vi "Measure DC 120629.vi"() -> ()   [LabVIEW 2011]
uses:
  Sub VIs/Trap cluster.ctl
  <vilib>/Utility/inputDevices.llb/closeKeyboard.vi
  <vilib>/Utility/inputDevices.llb/keyboardAcquire.vi
  <vilib>/Utility/file.llb/Write To Spreadsheet File (I64).vi
  <vilib>/vision/driver/NI_Vision_Acquisition_Software.lvlib
  <vilib>/vision/NI_Vision_Development_Module.lvlib
panel:
  in  "Apply Corrections":bool
  in  "View Licence":bool
  in  "ok":bool caption="Mark the center of \nthe spot using the \nzoom and the point\ntool, then click this \nbutton"
  in  "Stop program":bool
  in  "Updating trap cluster":bool
  out "Camera enabled":bool=TRUE
  out "SLM enabled":bool=TRUE
  in  "Run calibration":bool
  in  "Hologram generation":cluster{"Method":i32, "Iterations":i32}={"Method"=1, "Iterations"=50} {"Method" items=["Lenses & Gratings (3D)", " Gerchberg-Saxton (3D)", "Gerchberg-Saxton FFT (2D)"]}
  in  "Display hologram\nand computed \nimage plane":bool
  in  "ROI":T1={"Global Rectangle"=[39, 191, 388, 192], "Contours"=[{"Contour Type"=0, "ROI Type"=1, "Points"=[387, 191]}, {"Contour Type"=0, "ROI Type"=1, "Points"=[300, 191]}, {"Contour Type"=0, "ROI Type"=1, "Points"=[213, 191]}, {"Contour Type"=0, "ROI Type"=1, "Points"=[126, 191]}, {"Contour Type"=0, "ROI Type"=1, "Points"=[39, 191]}]}
  out "Image":T2(plugin-control)
  in  "Save\nHologram":bool
  in  "Image\naveraging":i32=100
  in  "?":bool
  in  "?":bool
  out "e desired":sgl=25.0
  out "timed out?":bool
  in  "Sync \nmeasurement":bool
  in  "images per \nhologram":i32=1
  in  "I step":dbl=0.05
  in  "Intensity path":bool
  in  "?":bool=TRUE
  out "Global Report":T3={"Mean Value"=0.014534721, "Standard Variation"=0.33891603, "Minimal Value"=0.0, "Maximal Value"=57.52, "Area (calibrated)"=1310720.0, "Area (pixels)"=1310720, "%"=100.0, "Calibration Valid"=TRUE} {"Mean Value" format="%.2f"; "%" format="%.2f"; "Area (calibrated)" format="%.2f"; "Maximal Value" format="%.2f"; "Minimal Value" format="%.2f"; "Standard Variation" format="%.2f"}
  in  "start path":path=path "E:/David/SLM characterization/Measured data/120420 - Trapping"
  in  "?":bool
  in  "s":bool=TRUE
  in  "Edit trap cluster":bool
  out "Lost Frames":u32
  in  "threshold":bool
  in  "Range":cluster{"Lower value":sgl, "Upper value":sgl}={"Lower value"=200.0, "Upper value"=4096.0} {"Upper value" format="%.2f"; "Lower value" format="%.2f"}
  in  "Display data":bool=TRUE
  in  "?":bool=TRUE
  in  "Purge data":bool
  in  "ROI size":dbl=44.0 min=2.0 step=2.0
  in  "Save data":bool
  in  "Video tracking":bool
  out "Calculated image plane":dbl[][](graph)
  out "Current trap pos":T4={"X (IMAQ)"=[451.25, 557.0, 662.75, 821.375, 874.25, 980.0, 1085.75], "Y (IMAQ)"=[588.5, 588.5, 588.5, 740.5156, 588.5, 588.5, 588.5], "Z"=[0.0, 0.0, 0.0, 0.0, 0.0, 0.0, 0.0], "I"=[0.0, 0.0, 0.0, 100.0, 100.0, 100.0, 0.0], "Trap number"=[0, 1, 2, 3, 4, 5, 6], "ROI number"=[0, 1, 2, 3, 4, 5, 6], "Number of traps"=7, "Group"=[FALSE, FALSE, FALSE, FALSE, FALSE, FALSE, FALSE]}
  out "NI Vision error":errorcluster
  out "CUDA/SLM error":errorcluster
  in  "Cancel calibration":bool
  in  "Skip step if \ntimed out":bool
  in  "Display path":bool=TRUE
  out "Average step time (ms)":dbl=61.852387843704776
  in  "Step time \n(ms)":u32=10
  in  "Pause":bool
  in  "cancel path":bool
  out "Step skipped":bool
  in  "Path controls":T5={"follow path"=FALSE, "Step length"=1.0, "Arrive \nsimultaneously"=TRUE, "Synchronize traps"=FALSE, "Add current \npositions to path"=FALSE}
  in  "Create path":bool
  out "Displayed Hologram":u8[][](graph)
  in  "Coordinate mapping \n(IMAQ to SLM)":T6={"cZ"=1.0, "cY"=0.3699422, "cX"=-0.3699422, "sZ"=0.0, "sY"=-181.0867, "sX"=244.71677}
  in  "Switch X/Y":bool
  in  "Max num of \nmeasurements":i32=-1
  # "Martin\nPersson 2011"
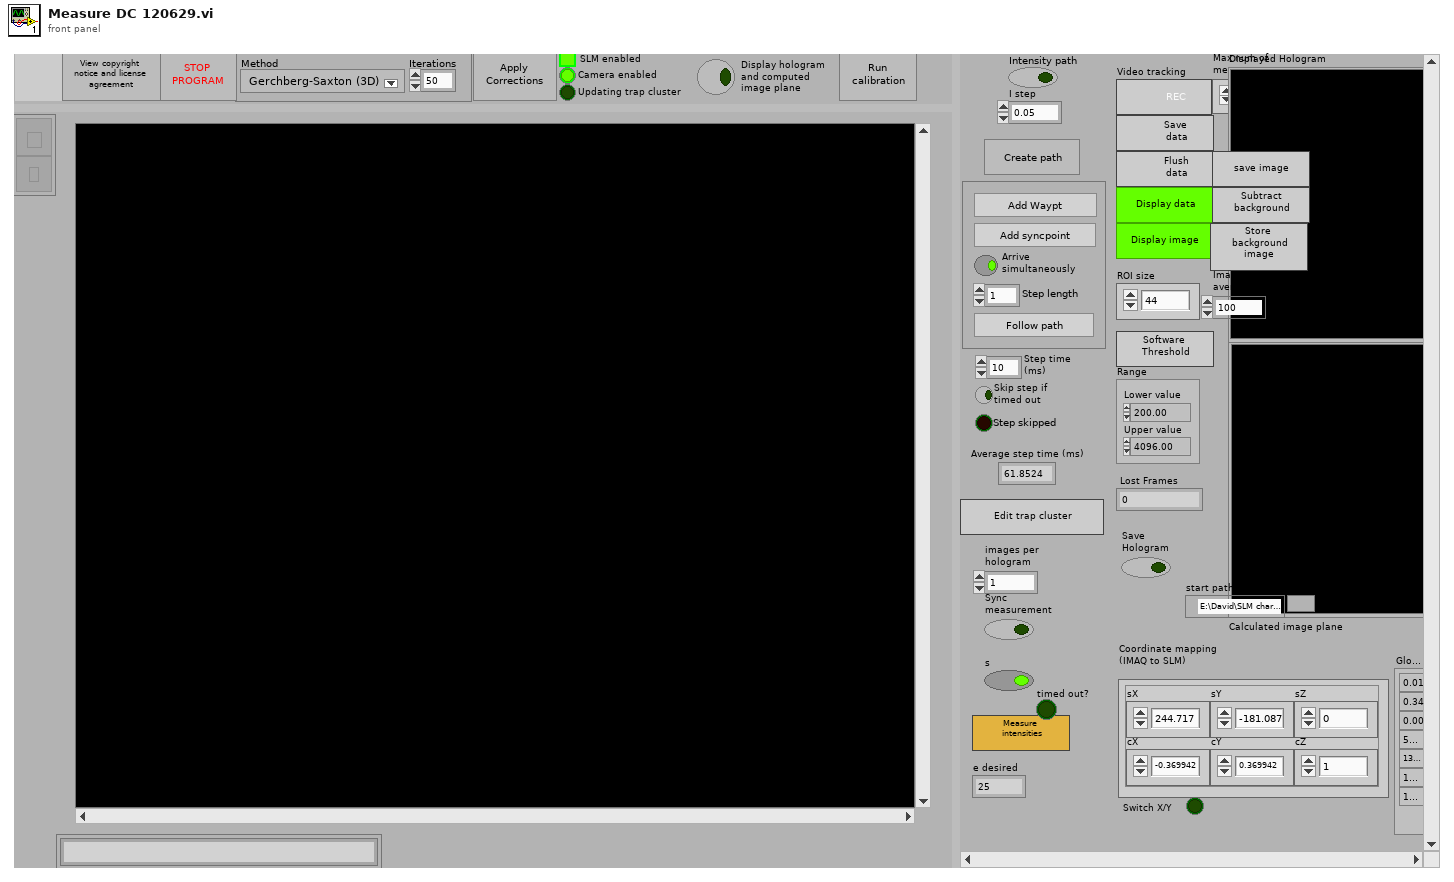
[diagram p1: front panel]
types:
  T1 = cluster{"Global Rectangle":i32[], "Contours":cluster{"Contour Type":u32, "ROI Type":u32, "Points":i32[]}[]}
  T2 = typedef "IMAQ Image.ctl" = refnum<image>
  T3 = cluster{"Mean Value":sgl, "Standard Variation":sgl, "Minimal Value":sgl, "Maximal Value":sgl, "Area (calibrated)":sgl, "Area (pixels)":u32, "%":sgl, "Calibration Valid":bool}
  T4 = typedef "Trap cluster.ctl" = cluster{"X (IMAQ)":sgl[], "Y (IMAQ)":sgl[], "Z":sgl[], "I":sgl[], "Trap number":i32[], "ROI number":i32[], "Number of traps":i32, "Group":bool[]}
  T5 = cluster{"follow path":bool, "Step length":dbl, "Arrive \nsimultaneously":bool, "Synchronize traps":bool, "Add current \npositions to path":bool}
  T6 = cluster{"cZ":sgl, "cY":sgl, "cX":sgl, "sZ":sgl, "sY":sgl, "sX":sgl}
  T7 = typedef "Image Type" = u32
  T8 = cluster{"CentroidX":dbl[], "CentroidY":dbl[], "I":dbl[], "Acquired Buffer Number":u32}
  T9 = typedef "IMAQdx.ctl" = refnum<k21>
  T10 = typedef "Rendezvous RefNum" = refnum<k1>
  T11 = enum16{"0", "1", "2", "3", "4", "5", "6", "7", "8", "9", "A", "B", "C", "D", "E", "F", "G", "H", "I", "J", "K", "L", "M", "N", "O", "P", "Q", "R", "S", "T", "U", "V", "W", "X", "Y", "Z", "F1", "F2", "F3", "F4", "F5", "F6", "F7", "F8", "F9", "F10", "F11", "F12", "F13", "F14", "F15", "ADD", "BACK", "BACKSLASH", "CAPITAL", "COMMA", "DECIMAL", "DELETE", "DIVIDE", "DOWN", "END", "EQUALS", "ESCAPE", "GRAVE (`)", "HOME", "INSERT", "LBRACKET", "LCONTROL", "LEFT", "L ALT", "LSHIFT", "LWIN", "MINUS", "MULTIPLY", "NEXT", "NUMLOCK", "NUMPAD_0", "NUMPAD_1", "NUMPAD_2", "NUMPAD_3", "NUMPAD_4", "NUMPAD_5", "NUMPAD_6", "NUMPAD_7", "NUMPAD_8", "NUMPAD_9", "PAUSE", "PERIOD", "PRIOR (PG UP)", "RBRACKET", "RCONTROL", "RETURN", "RIGHT", "R ALT", "RSHIFT", "RWIN", "SCROLL", "SEMICOLON", "SLASH", "SPACE", "SUBTRACT", "TAB", "UP", "ENTER (num pad)", "' (quote)"}[]
  T12 = typedef "LVRectTypeDef.ctl" = cluster{"left":i16, "top":i16, "right":i16, "bottom":i16}
  T13 = cluster{"output cluster 2":cluster{"CentroidX":dbl[], "CentroidY":dbl[], "I":dbl[], "Acquired Buffer Number":u32}, "output cluster 2":T4}[]
  T14 = cluster{"CentroidX":dbl[], "CentroidY":dbl[], "I":dbl[], "Acquired Buffer Number":u32}[]
  T15 = cluster{"output cluster 2":cluster{"CentroidX":dbl[], "CentroidY":dbl[], "I":dbl[], "Acquired Buffer Number":u32}, "output cluster 2":T4}
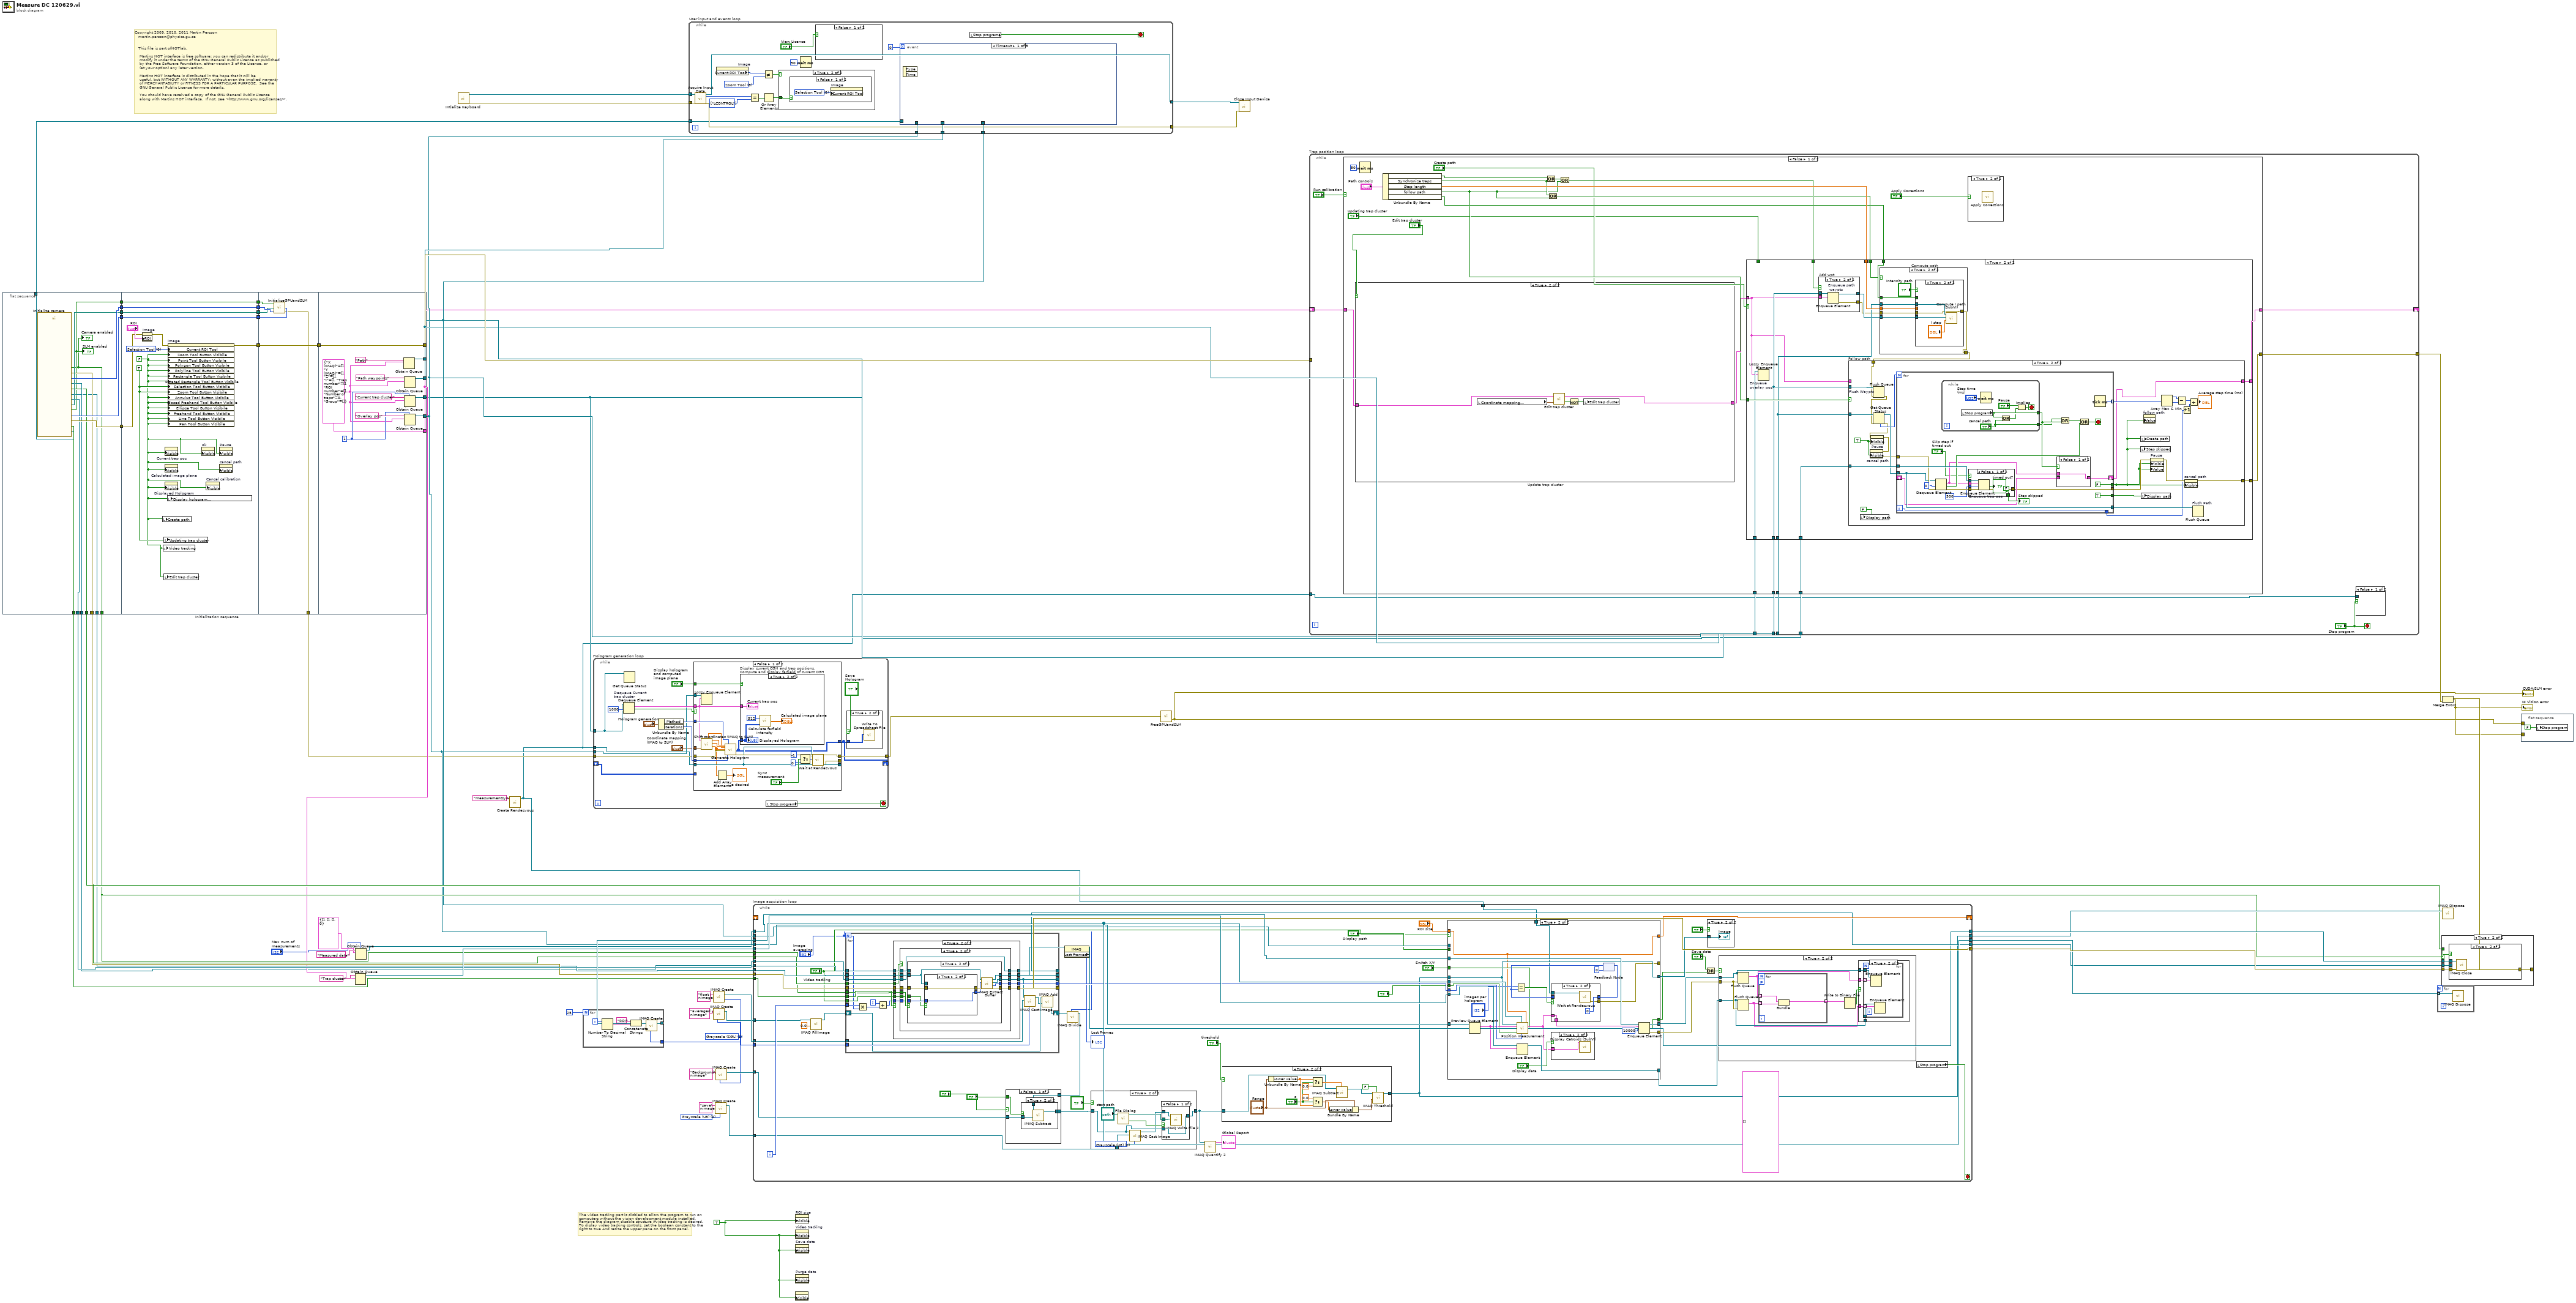
[diagram p0: block diagram]
diagram:
  w2 = T7 0 items=["Grayscale (U8)", "Grayscale (I16)", "Grayscale (SGL)", "Complex (CSG)", "RGB (U32)", "HSL (U32)", "RGB (U64)", "Grayscale (U16)"] ("Image Type")
  w4 = T7 2 items=["Grayscale (U8)", "Grayscale (I16)", "Grayscale (SGL)", "Complex (CSG)", "RGB (U32)", "HSL (U32)", "RGB (U64)", "Grayscale (U16)"] ("Image Type")
  w49 = TRUE ("Visible")
  # "Copyright 2009, 2010, 2011 Martin Persson \n   martin.persson@physics.gu.se\n\n\n   This file is part ofHOTlab.\n\n    Martins HOT interface is free software: you can redistribute it and/or \n    modify it under the terms of the GNU General Public License as published \n    by the Free Software Foundation, either version 3 of the License, or\n    (at your option) any later version.\n\n    Martins HOT interface is distributed in the hope that it will be \n    useful, but WITHOUT ANY WARRANTY; without even the implied warranty\n    of MERCHANTABILITY or FITNESS FOR A PARTICULAR PURPOSE.  See the\n    GNU General Public License for more details.\n\n    You should have received a copy of the GNU General Public License\n    along with Martins HOT interface.  If not, see <http://www.gnu.org/licenses/>."
  # "The video tracking part is disbled to allow the program to run on\ncomputers without the vision development module installed. \nRemove the diagram disable structure ifvideo tracking is desired. \nTo diplay video tracking controls, set the boolean constant to the \nright to true And resize the upper pane on the front panel."
  n1 = flat-sequence "Initialization sequence" {
    tunnel: [w65] -> w41
    tunnel: [w74] -> w40
    tunnel: [w73] -> w39
    tunnel: [w72] -> w38
    tunnel: [w71] -> w37
    tunnel: [w70] -> w17
    tunnel: [w69] -> w35
    tunnel: [w68] -> w34
    tunnel: [w67] -> w33
    tunnel: [w66] -> w32
    tunnel: [w64] -> w31
    tunnel: [w63] -> w18
    tunnel: [w62] -> w16
    tunnel: w41 -> [w82]
    tunnel: w40 -> [w80]
    tunnel: w39 -> [w85]
    tunnel: w38 -> [w84]
    tunnel: w37 -> [w83]
    tunnel: [w82] -> w26
    tunnel: [w77] -> w25
    tunnel: [w85] -> w23
    tunnel: [w84] -> w22
    tunnel: [w83] -> w21
    tunnel: w26 -> [w88]
    tunnel: w25 -> [w91]
    tunnel: [w91] -> w24
    tunnel: w23 -> [w89]
    tunnel: w22 -> [w90]
    tunnel: w21 -> [w87]
    tunnel: [w86] -> w20
    tunnel: [w102] -> w36
    tunnel: w24 -> [w102]
    tunnel: [w100] -> w30
    tunnel: [w98] -> w29
    tunnel: [w96] -> w19
    tunnel: [w95] -> w28
    tunnel: [w92] -> w27
    frame #0 {
      n2 = call "Initialize camera.vi"() -> ("CUDA device ID"=w72:i32, "IMAQdx Session Out"=w69:T9, "TrueFrame out"=w73:i32, "IMAQ camera"=w67:bool, "Image buffers"=w62:T2[], "Image reference out"=w70:T2, "Ring?"=w63:bool, "SLM enabled"=w65:bool, "Camera enabled"=w64:bool, "Vision error out"=w74:errorcluster, "LUT path out"=w71:path, "IMAQ Session Out"=w66:refnum<k11>, "Camera error"=w68:errorcluster)  [unwired: 3 in]
      "Camera enabled" <- w64
      "SLM enabled" <- w65
    }
    frame #1 {
      w76 = TRUE ("ROI Tool Buttons Visibile:Zoom Tool Button Visible")
      w75 = FALSE ("ROI Tool Buttons Visibile:Zoom Tool Button Visible")
      w79 = u32 0 items=["Zoom Tool"=8, "Selection Tool"=0, "Pan Tool"=9, "Point Tool"=1, "Line Tool"=2, "Rectangle Tool"=3, "Rotated Rectangle Tool"=12, "Polyline Tool"=10, "Polygon Tool"=5, "Freehand Tool"=11, "Closed Freehand Tool"=6, "Ellipse Tool"=4, "Annulus Tool"=7] ("Current ROI Tool")
      n3 = property on="Image" class="ImageControl"(error in=w80, "ROI"="ROI") -> (error out=w78:errorcluster)  [unwired: 1 in, 1 out]
      n4 = local write "Create path"(w75) -> ()
      n5 = local write "Video tracking"(w75) -> ()
      n6 = local write "Updating trap cluster"(w76) -> ()
      n7 = local write "Edit trap cluster"(w75) -> ()
      n8 = property on="Current trap pos" class="Clust (strict)"("Visible"=w75) -> ()  [unwired: 2 in, 2 out]
      n9 = property on="Calculated image plane" class="IntGraph (strict)"("Visible"=w75) -> ()  [unwired: 2 in, 2 out]
      n10 = property on="Displayed Hologram" class="IntGraph (strict)"("Visible"=w75) -> ()  [unwired: 2 in, 2 out]
      n11 = local write "Display hologram\nand computed \nimage plane"(w75) -> ()
      n12 = property on="Image" class="ImageControl"(error in=w78, "Current ROI Tool"=w79, "Zoom Tool Button Visibile"=w75, "Point Tool Button Visibile"=w75, "Polygon Tool Button Visibile"=w75, "Polyline Tool Button Visibile"=w75, "Rectangle Tool Button Visibile"=w75, "Rotated Rectangle Tool Button Visibile"=w75, "Selection Tool Button Visibile"=w76, "Zoom Tool Button Visibile"=w76, "Annulus Tool Button Visibile"=w75, "Closed Freehand Tool Button Visibile"=w75, "Ellipse Tool Button Visibile"=w75, "Freehand Tool Button Visibile"=w75, "Line Tool Button Visibile"=w75, "Pan Tool Button Visibile"=w75) -> (error out=w77:errorcluster)  [unwired: 1 in, 1 out]
      n13 = property on="ok" class="Bool"("Visible"=w75) -> ()  [unwired: 2 in, 2 out]
      n14 = property on="Cancel calibration" class="Bool"("Visible"=w75) -> ()  [unwired: 2 in, 2 out]
      n15 = property on="Pause" class="Bool (strict)"("Visible"=w75) -> ()  [unwired: 2 in, 2 out]
      n16 = property on="cancel path" class="Bool"("Visible"=w75) -> ()  [unwired: 2 in, 2 out]
    }
    frame #2 {
      n17 = call "InitializeGPUandSLM.vi"("TrueFrame"=w89, "deviceId"=w90, "Path to LUT file"=w87, "SLM enabled"=w88) -> ("CUDA/SLM error"=w86:errorcluster)  [unwired: 1 out]
    }
    frame #3 {
      w93 = 1 ("max queue size (-1, unlimited)")
      w92 = T4 {"X (IMAQ)"=[], "Y (IMAQ)"=[], "Z"=[], "I"=[], "Trap number"=[], "ROI number"=[], "Number of traps"=0, "Group"=[]} ("output cluster 2")
      n18 = Obtain Queue(name (unnamed)="Path", element data type=w92) -> (queue out=w100:refnum<queue>)  [unwired: 3 in, 2 out]
      n19 = Obtain Queue(name (unnamed)="Path waypoints", element data type=w92) -> (queue out=w98:refnum<queue>)  [unwired: 3 in, 2 out]
      n20 = Obtain Queue(max queue size (-1, unlimited)=w93, name (unnamed)="Current trap cluster", element data type=w92) -> (queue out=w96:refnum<queue>)  [unwired: 2 in, 2 out]
      n21 = Obtain Queue(max queue size (-1, unlimited)=w93, name (unnamed)="Overlay pos", element data type=w92) -> (queue out=w95:refnum<queue>)  [unwired: 2 in, 2 out]
    }
  }
  n22 = Obtain Queue(name (unnamed)="Trap cluster", element data type=w27) -> (queue out=w54:refnum<queue>)  [unwired: 3 in, 2 out]
  n23 = Obtain Queue(max queue size (-1, unlimited)="Max num of \nmeasurements", name (unnamed)="Measured data", element data type=T8 {"CentroidX"=[], "CentroidY"=[], "I"=[], "Acquired Buffer Number"=0} ("output cluster 2")) -> (queue out=w13:refnum<queue>)  [unwired: 2 in, 2 out]
  n24 = call <vilib>:"Intialize Keyboard.vi"() -> ("error out"=w43:errorcluster, "device ID"=w61:refnum<k1>)  [unwired: 1 in, 9 out]
  n25 = call <vilib>:"Create Rendezvous.vi"("name (unnamed)"="measurementsync") -> ("rendezvous"=w11:T10)  [unwired: 4 in, 2 out]
  n26 = for {
    N: 25 -> [_]
    tunnel: [w108] -> w58 mode=indexing
    tunnel: w4 -> [w103]
    i -> [w105]
    n27 = Number To Decimal String(number=w105) -> (decimal integer string=w104:string)  [unwired: 1 in]
    n28 = Concatenate Strings("ROI" ("Image Name"), w104) -> (w106:string)
    n29 = call "IMAQ Create"("Image Name"=w106, "Image Type"=w103) -> ("New Image"=w108:T2)  [unwired: 3 in, 1 out]
  }
  n30 = while "Hologram generation loop" {
    tunnel: w19 -> [w112]
    tunnel: w28 -> [w121]
    tunnel: w20 -> [w116]
    tunnel: [w115] -> w14
    tunnel: w11 -> [w114]
    shift-right: [w111] -> _
    shift-left: _ -> [w110]
    stop <- w113 stop-if-true
    n31 = Dequeue Element "Dequeue Current \ntrap cluster"(queue=w112, timeout in ms (-1)=1000) -> (element=w122:T4, timed out?=w120:bool)  [unwired: 1 in, 2 out]
    n32 = Get Queue Status(queue=w112) -> ()  [unwired: 2 in, 8 out]
    n33 = Unbundle By Name("Hologram generation") -> ("Method"=w125:i32, "Iterations"=w124:i32)
    n34 = case shown="False" w120 {
      tunnel: "Coordinate mapping \n(IMAQ to SLM)" -> [w146 _]
      tunnel: "Display hologram\nand computed \nimage plane" -> [w139 _]
      tunnel: w125 -> [w142 _]
      tunnel: w124 -> [w141 _]
      tunnel: w122 -> [w136 _]
      tunnel: w121 -> [w140 _]
      tunnel: w116 -> [w138 w153]
      tunnel: [w137 w153] -> w115
      tunnel: w114 -> [w131 w152]
      tunnel: [w131 w152] -> _
      tunnel: [w130 _] -> _
      tunnel: [w127 w151] -> w111
      tunnel: w110 -> [_ w151]
      frame False {
        n35 = Lossy Enqueue Element(queue=w140, element=w136) -> ()  [unwired: 1 in, 4 out]
        n36 = call "Shift coordinates (IMAQ to SLM).vi"("Trap cluster"=w136, "Coordinate mapping \n(IMAQ to SLM)"=w146) -> ("X (SLM)"=w143:sgl[], "Y (SLM)"=w145:sgl[], "Intensities"=w129:sgl[], "Z (SLM)"=w144:sgl[])  [unwired: 1 in, 1 out]
        n37 = Add Array Elements(numeric array=w129) -> (sum=→"e desired":sgl)
        n38 = call "Generate Hologram.vi"("x"=w143, "y"=w145, "z"=w144, "spot_intensities"=w129, "CUDA/SLM error in"=w138, "N_iterations"=w141, "method"=w142) -> ("CGH out"=w127:u8[][], "CUDA/SLM error out"=w137:errorcluster)  [unwired: 17 in, 2 out]
        n39 = case "Display current CGH and trap positions.\nCompute and display farfield of current CGH" shown="True" w139 {
          tunnel: w127 -> [_ w149]
          tunnel: w136 -> [_ w147]
          frame False {
          }
          frame True {
            n40 = call "Calculate farfield intensity.vi"("h_pSLM"=w149, "SLMsize"=512 ("Numeric")) -> ("Calculated image plane"=→"Calculated image plane":dbl[][])
            "Displayed Hologram" <- w149
            "Current trap pos" <- w147
          }
        }
        n41 = Select(t=-1 ("ms timeout (-1)"), s="Sync \nmeasurement", f=0) -> (s? t:f=w133:i32)
        n42 = call <vilib>:"Wait at Rendezvous.vi"("ms timeout (-1)"=w133, "rendezvous"=w131) -> ("error out"=w130:errorcluster)  [unwired: 3 in, 2 out]
      }
      frame True {
      }
    }
    n43 = local read "Stop program"() -> (w113:bool)
    n44 = case shown="True" "Save\nHologram" {
      tunnel: w111 -> [_ w126]
      frame False {
      }
      frame True {
        n45 = call-poly <vilib>:"Write To Spreadsheet File.vi"("2D data"=w126) -> ()  [unwired: 7 in, 1 out]
      }
    }
  }
  n46 = while "User input and events loop" {
    tunnel: w61 -> [w172]
    tunnel: w28 -> [w161]
    tunnel: w29 -> [w160]
    tunnel: w30 -> [w159]
    tunnel: [w158] -> w44
    tunnel: w43 -> [w157]
    tunnel: [w156] -> w42
    tunnel: w16 -> [w154]
    stop <- w164 stop-if-true
    w169 = u32 8 items=["Zoom Tool"=8, "Selection Tool"=0, "Pan Tool"=9, "Point Tool"=1, "Line Tool"=2, "Rectangle Tool"=3, "Rotated Rectangle Tool"=12, "Polyline Tool"=10, "Polygon Tool"=5, "Freehand Tool"=11, "Closed Freehand Tool"=6, "Ellipse Tool"=4, "Annulus Tool"=7] ("Current ROI Tool")
    w166 = T11 [enum."LCONTROL"] items=["0", "1", "2", "3", "4", "5", "6", "7", "8", "9", "A", "B", "C", "D", "E", "F", "G", "H", "I", "J", "K", "L", "M", "N", "O", "P", "Q", "R", "S", "T", "U", "V", "W", "X", "Y", "Z", "F1", "F2", "F3", "F4", "F5", "F6", "F7", "F8", "F9", "F10", "F11", "F12", "F13", "F14", "F15", "ADD", "BACK", "BACKSLASH", "CAPITAL", "COMMA", "DECIMAL", "DELETE", "DIVIDE", "DOWN", "END", "EQUALS", "ESCAPE", "GRAVE (`)", "HOME", "INSERT", "LBRACKET", "LCONTROL", "LEFT", "L ALT", "LSHIFT", "LWIN", "MINUS", "MULTIPLY", "NEXT", "NUMLOCK", "NUMPAD_0", "NUMPAD_1", "NUMPAD_2", "NUMPAD_3", "NUMPAD_4", "NUMPAD_5", "NUMPAD_6", "NUMPAD_7", "NUMPAD_8", "NUMPAD_9", "PAUSE", "PERIOD", "PRIOR (PG UP)", "RBRACKET", "RCONTROL", "RETURN", "RIGHT", "R ALT", "RSHIFT", "RWIN", "SCROLL", "SEMICOLON", "SLASH", "SPACE", "SUBTRACT", "TAB", "UP", "ENTER (num pad)", "' (quote)"] ("keys pressed")
    n47 = call-poly <vilib>:"Acquire Input Data.vi"("device ID"=w172, "error in (no error)"=w157) -> ("device ID"=w158:refnum<k1>, "keys pressed"=w165:T11, "error out"=w156:errorcluster)  [unwired: 15 out]
    n48 = property on="Image" class="ImageControl"() -> ("Current ROI Tool"=w168:u32)  [unwired: 2 in, 2 out]
    n49 = Equal?(x=w165, y=w166) -> (x = y?=w167:bool[])
    n50 = Not Equal?(x=w168, y=w169) -> (x != y?=w170:bool)
    n51 = Or Array Elements(Boolean array=w167) -> (logical OR=w171:bool)
    n52 = case shown="True" w170 {
      tunnel: w171 -> [_ w206]
      frame False {
      }
      frame True {
        n53 = case shown="False" w206 {
          frame False {
            w207 = u32 0 items=["Zoom Tool"=8, "Selection Tool"=0, "Pan Tool"=9, "Point Tool"=1, "Line Tool"=2, "Rectangle Tool"=3, "Rotated Rectangle Tool"=12, "Polyline Tool"=10, "Polygon Tool"=5, "Freehand Tool"=11, "Closed Freehand Tool"=6, "Ellipse Tool"=4, "Annulus Tool"=7] ("Current ROI Tool")
            n54 = property on="Image" class="ImageControl"("Current ROI Tool"=w207) -> ()  [unwired: 2 in, 2 out]
          }
          frame True {
            w208 = u32 1 items=["Zoom Tool"=8, "Selection Tool"=0, "Pan Tool"=9, "Point Tool"=1, "Line Tool"=2, "Rectangle Tool"=3, "Rotated Rectangle Tool"=12, "Polyline Tool"=10, "Polygon Tool"=5, "Freehand Tool"=11, "Closed Freehand Tool"=6, "Ellipse Tool"=4, "Annulus Tool"=7] ("Current ROI Tool")
            n55 = property on="Image" class="ImageControl"("Current ROI Tool"=w208) -> ()  [unwired: 2 in, 2 out]
          }
        }
      }
    }
    n56 = Wait (ms)(milliseconds to wait=u32 50) -> ()  [unwired: 1 out]
    n57 = case shown="False" "View Licence" {
      frame False {
      }
      frame True {
        n58 = call "View license.vi"() -> ()  [unwired: 1 in]
      }
    }
    n59 = event shown="[0] Timeout" {
      selector: _ -> [_ _ _ _ _ _ _ _ _]
      dyn-events: _ -> [_ _ _ _ _ _ _ _ _]
      timeout: 0 -> [_ _ _ _ _ _ _ _ _]
      tunnel: w161 -> [_ _ w183 _ _ _ _ _ _]
      tunnel: w160 -> [_ _ w182 _ _ _ _ _ _]
      tunnel: w159 -> [_ _ w186 _ _ _ _ _ _]
      tunnel: w154 -> [_ _ _ _ _ _ w198 _ _]
      event Timeout {
        n60 = event-data() -> ()  [unwired: 1 in, 2 out]
      }
      event "Display hologram\nand computed \nimage plane": Value Change {
        n61 = event-data() -> ("NewVal"=w174:bool)  [unwired: 1 in, 4 out]
        n62 = property on="Current trap pos" class="Clust (strict)"("Visible"=w174) -> ()  [unwired: 2 in, 2 out]
        n63 = property on="Displayed Hologram" class="IntGraph (strict)"("Visible"=w174) -> ()  [unwired: 2 in, 2 out]
        n64 = property on="Calculated image plane" class="IntGraph (strict)"("Visible"=w174) -> ()  [unwired: 2 in, 2 out]
        n65 = property on="Property Node" class="VI"() -> ("Front Panel.WinBounds"=w181:T12)  [unwired: 2 in, 2 out]
        n66 = Unbundle By Name(w181) -> ("right"=w180:i16, "left"=w179:i16)
        n67 = Subtract(x=w180, y=w179) -> (x-y=w178:i16)
        n68 = Select(t=i16 500 ("x-y"), s=w174, f=i16 196 ("x-y")) -> (s? t:f=w173:i16)
        n69 = Subtract(x=w178, y=w173) -> (x-y=w177:i16)
        n70 = property on="Splitter" class="Splitter"("Position"=w177) -> ()  [unwired: 2 in, 2 out]
      }
      event "Create path": Value Change {
        n71 = event-data() -> ()  [unwired: 1 in, 5 out]
        n72 = property on="follow path" class="Bool (strict)"("Value"=FALSE) -> ()  [unwired: 2 in, 2 out]
        n73 = Flush Queue "Flush path \nwaypt queue"(queue=w182) -> ()  [unwired: 1 in, 3 out]
        n74 = Preview Queue Element(queue=w183) -> (element=w184:T4, error out=w187:errorcluster)  [unwired: 2 in, 2 out]
        n75 = Flush Queue "Flush path queue"(queue=w186) -> (queue out=w185:refnum<queue>)  [unwired: 1 in, 2 out]
        n76 = Enqueue Element "Enqueue current \ntrap pos in path"(queue=w185, element=w184) -> ()  [unwired: 2 in, 3 out]
        n77 = Enqueue Element "Enqueue current \ntrap pos in path \nwaypts"(queue=w182, element=w184, error in (no error)=w187) -> ()  [unwired: 1 in, 3 out]
      }
      event "cancel path": Value Change {
        n78 = event-data() -> ()  [unwired: 1 in, 5 out]
        n79 = local write "Create path"(FALSE ("Visible")) -> ()
      }
      event "Image", "Coordinate mapping \n(IMAQ to SLM)": Mouse Down {
        w190 = FALSE ("Edit trap cluster")
        n80 = event-data() -> ()  [unwired: 1 in, 7 out]
        n81 = local write "Updating trap cluster"(TRUE ("Update trap positions")) -> ()
        n82 = local write "Edit trap cluster"(w190) -> ()
        n83 = call <vilib>:"Application Directory.vi"() -> ("Application Directory"=w191:path)
        n84 = Build Path(base path=w191, name or relative path="Sub VIs\\Edit trap cluster.vi") -> (appended path=w194:path)
        n85 = Open VI Reference(vi path=w194) -> (vi reference=w193:refnum<vi>)  [unwired: 5 in, 1 out]
        n86 = property class="VI"(reference=w193, "Front Panel.Open"=w190) -> ()  [unwired: 1 in, 2 out]
      }
      event "Image", "Coordinate mapping \n(IMAQ to SLM)": Mouse Up {
        n87 = event-data() -> ()  [unwired: 1 in, 7 out]
        n88 = flat-sequence {
          frame #0 {
            n89 = Wait (ms)(milliseconds to wait=u32 100) -> ()  [unwired: 1 out]
          }
          frame #1 {
            n90 = local write "Updating trap cluster"(FALSE ("Update trap positions")) -> ()
          }
        }
      }
      event "Video tracking": Value Change {
        n91 = event-data() -> ()  [unwired: 1 in, 5 out]
        n92 = for {
          tunnel: w198 -> [w199] mode=indexing
          n93 = call "IMAQ Clear Overlay"("Image"=w199) -> ()  [unwired: 9 in, 2 out]
        }
      }
      event "Display data": Value Change {
        n94 = event-data() -> ("NewVal"=w201:bool)  [unwired: 1 in, 4 out]
        n95 = call <vilib>:"Application Directory.vi"() -> ("Application Directory"=w200:path)
        n96 = Build Path(base path=w200, name or relative path="Sub VIs\\Display Cetroids (SubVI).vi") -> (appended path=w204:path)
        n97 = Open VI Reference(vi path=w204) -> (vi reference=w203:refnum<vi>)  [unwired: 5 in, 1 out]
        n98 = property class="VI"(reference=w203, "Front Panel.Open"=w201) -> ()  [unwired: 1 in, 2 out]
      }
      event "Edit trap cluster": Value Change {
        n99 = event-data() -> ("NewVal"=w205:bool)  [unwired: 1 in, 4 out]
        n100 = local write "Updating trap cluster"(w205) -> ()
      }
    }
    n101 = local read "Stop program"() -> (w164:bool)
  }
  n102 = call "IMAQ Create"("Image Name"="averaged \nimage", "Image Type"=w4) -> ("New Image"=w5:T2)  [unwired: 3 in, 1 out]
  n103 = call "IMAQ Create"("Border Size"=w4, "Image Name"="float \nimage") -> ("New Image"=w9:T2)  [unwired: 3 in, 1 out]
  n104 = call "IMAQ Create"("Image Name"="save\nimage", "Image Type"=w2) -> ("New Image"=w1:T2)  [unwired: 3 in, 1 out]
  n105 = call "IMAQ Create"("Image Name"="Background\nimage", "Image Type"=w4) -> ("New Image"=w7:T2)  [unwired: 3 in, 1 out]
  n106 = while "Image acquisition loop" {
    tunnel: w31 -> [w240]
    tunnel: w17 -> [w261]
    tunnel: w32 -> [w260]
    tunnel: [w237] -> w60
    tunnel: [w259] -> w59
    tunnel: w58 -> [w253]
    tunnel: w13 -> [w257]
    shift-right: [w256] -> _
    shift-left: _ -> [_]
    tunnel: w54 -> [w255]
    tunnel: [w253] -> w52
    tunnel: [w233] -> w51
    tunnel: [w252] -> w50
    tunnel: w35 -> [w251]
    tunnel: w33 -> [w250]
    tunnel: w28 -> [w249]
    tunnel: w30 -> [w248]
    tunnel: w34 -> [w246]
    tunnel: w18 -> [w236]
    tunnel: w11 -> [w224]
    tunnel: w4 -> [w219]
    tunnel: w9 -> [w218]
    tunnel: w7 -> [w216]
    tunnel: w5 -> [w212]
    tunnel: w1 -> [w209]
    i -> [w225]
    stop <- w258 stop-if-true
    (unwired) T13 [] ("Array")
    n107 = call "IMAQ FillImage"("Pixel Value (U8, U16, I16, Float)"=sgl 0.0, "Image"=w212) -> ("Image Out"=w211:T2)  [unwired: 8 in, 1 out]
    n108 = for {
      N: "Image\naveraging" -> [w281]
      tunnel: w261 -> [w295]
      tunnel: w260 -> [w294]
      tunnel: [w293] -> w259
      tunnel: [w292] -> w252
      tunnel: w251 -> [w291]
      tunnel: w250 -> [w290]
      tunnel: w246 -> [w289]
      tunnel: [w288] -> w245
      tunnel: w240 -> [w287]
      tunnel: w236 -> [w286]
      tunnel: [w285] -> w235
      tunnel: "Video tracking" -> [w284]
      tunnel: [w278] -> _
      tunnel: w225 -> [w283]
      tunnel: w219 -> [w276]
      tunnel: w218 -> [w275]
      shift-right: [w277] -> w221
      shift-left: w211 -> [w274]
      i -> [w279]
      n109 = Multiply(x=w283, y=w281) -> (x*y=w282:i32)
      n110 = Add(x=w279, y=w282) -> (x+y=w280:i32)
      n111 = case shown="True" w287 {
        tunnel: w295 -> [w298 w312]
        tunnel: w294 -> [w297 w311]
        tunnel: [w297 w310] -> w285
        tunnel: [w296 w309] -> w293
        tunnel: [w298 w308] -> w278
        tunnel: [w299 w307] -> w292
        tunnel: w291 -> [w299 w306]
        tunnel: w290 -> [_ w305]
        tunnel: w289 -> [w296 w304]
        tunnel: [_ w303] -> w288
        tunnel: w286 -> [_ w302]